vi "FRC ADI MXP IMU Example.vi"() -> ()   [LabVIEW 2015]
doc: "SimpleGyro Example\n\nThis example shows how to use a SimpleGyro sensor connected to the SPI port on the RoboRIO.\n\nThis example expects a USB cable connected from your development PC to the Type B USB Jack (next to the power input) on the roboRIO."
uses:
  <vilib>/Rock Robotics/SystemInterfaces/spilib/spi_bus.ctl
  ADI MXP IMU/FRC ADI MXP IMU.lvlib
panel:
  in  "AHRS Yaw Axis":enum16{"X", "Y", "Z"}(ring)=enum."Z"
  out "Sensor Ready?":bool
  out "IMU AHRS Delta":cluster{"Pitch":dbl, "Roll":dbl, "Yaw":dbl}
  out "IMU AHRS":cluster{"Pitch":dbl, "Roll":dbl, "Yaw":dbl}
  out "RAW IMU Data":T1
  out "IMU Angle Delta":cluster{"X":dbl, "Y":dbl, "Z":dbl}
  in  "Reset Angles?":bool
  out "Device Found?":bool
  in  "stop":bool
  # "FRC Analog Devices ADIS16448 IMU Example"
  # "FRC ADI MXP Placement"
  # "Raw IMU Output Data"
  # "IMU Deltas"
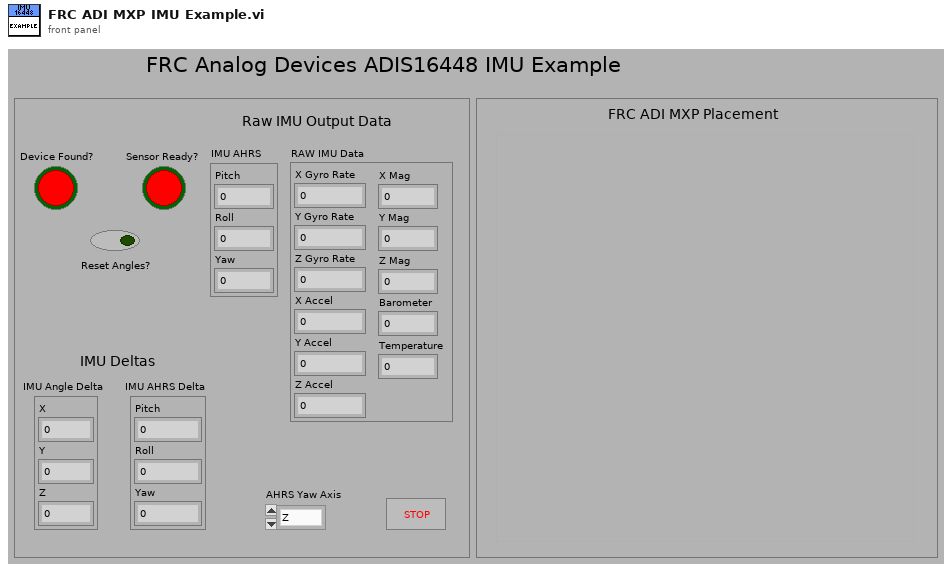
[diagram p1: front panel]
types:
  T1 = cluster{"X Gyro Rate":dbl, "Y Gyro Rate":dbl, "Z Gyro Rate":dbl, "X Accel":dbl, "Y Accel":dbl, "Z Accel":dbl, "X Mag":dbl, "Y Mag":dbl, "Z Mag":dbl, "Barometer":dbl, "Temperature":dbl}
  T2 = typedef "spi_bus.ctl" = enum16{"SPI On-Board, CS0", "SPI On-Board, CS1", "SPI On-Board, CS2", "SPI On-Board, CS3", "SPI MXP", "Invalid"}
  T3 = typedef "FRC ADI MXP IMU.lvlib/WPI_AnalogDevicesIMUInterruptDevRef.ctl" = cluster{"SimpleGyroDevRef":T4, "InterruptRef":T5}
  T4 = typedef "FRC ADI MXP IMU.lvlib/WPI_AnalogDevicesIMUDevRef.ctl" = cluster{"DevStatus":errorcluster, "Handle":i32, "SPI Bus":T2, "Device Found":bool, "Sample Rate":dbl, "Device Ready":bool, "Yaw Axis":enum16{"X", "Y", "Z"}}
  T5 = typedef "WPI_InterruptRef.ctl" = cluster{"DevStatus":errorcluster, "InterruptIndex":T6}
  T6 = typedef "FPGA_InterruptIndex.ctl" = enum8{"0", "1", "2", "3", "4", "5", "6", "7", "Invalid"}
  T7 = cluster{"X Angle":dbl, "Y Angle":dbl, "Z Angle":dbl}
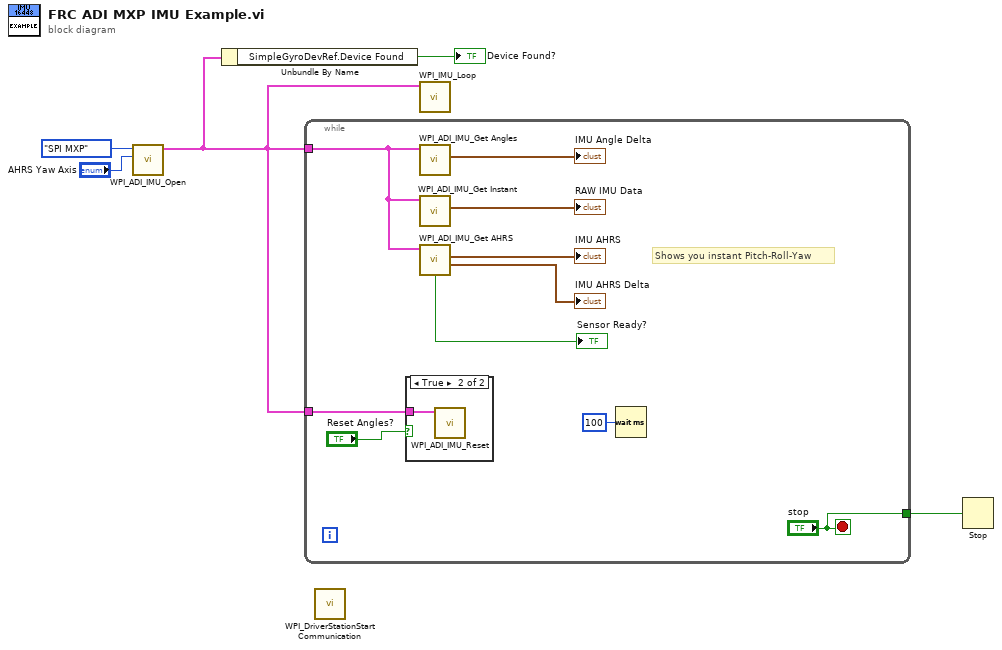
[diagram p0: block diagram]
diagram:
  n1 = call "WPI_ADI_IMU_Open.vi"("Yaw Axis"="AHRS Yaw Axis", "SPI Chip Select"=spi_bus."SPI MXP") -> ("ADI IMU Interrupt DevRef"=w2:T3)  [unwired: 8 in, 1 out]
  n2 = Unbundle By Name(w2) -> ("SimpleGyroDevRef.Device Found"=→"Device Found?":bool)
  n3 = while {
    tunnel: w2 -> [w7]
    tunnel: ["stop"] -> w4
    tunnel: w2 -> [w14]
    stop <- "stop" stop-if-true
    # "Shows you instant Pitch-Roll-Yaw"
    n4 = case shown="True" "Reset Angles?" {
      tunnel: w14 -> [_ w16]
      frame False {
      }
      frame True {
        n5 = call "WPI_ADI_IMU_Reset.vi"("ADI IMU Interrupt DevRef"=w16) -> ()  [unwired: 9 in, 2 out]
      }
    }
    n6 = call "WPI_ADI_IMU_Get Angles.vi"("ADI IMU Interrupt DevRef"=w7) -> ("IMU Angles"=→"IMU Angle Delta":T7)  [unwired: 7 in, 3 out]
    n7 = call "WPI_ADI_IMU_Get Instant.vi"("ADI IMU Interrupt DevRef"=w7) -> ("IMU Data"=→"RAW IMU Data":T1)  [unwired: 7 in, 3 out]
    n8 = call "WPI_ADI_IMU_Get AHRS.vi"("ADI IMU Interrupt DevRef"=w7) -> ("IMU AHRS DELTA"=→"IMU AHRS Delta":cluster{"Pitch":dbl, "Roll":dbl, "Yaw":dbl}, "IMU AHRS"=→"IMU AHRS":cluster{"Pitch":dbl, "Roll":dbl, "Yaw":dbl}, "Sensor Ready Out"=→"Sensor Ready?":bool)  [unwired: 6 in, 2 out]
    n9 = Wait (ms)(milliseconds to wait=u32 100) -> ()  [unwired: 1 out]
  }
  n10 = call <vilib>:"WPI_DriverStationStart Communication.vi"() -> ()  [unwired: 12 in]
  n11 = call "WPI_IMU_Loop.vi"("ADI IMU Interrupt DevRef"=w2) -> ()  [unwired: 10 in, 1 out]
  n12 = Stop(stop? (T)=w4) -> ()
